vi "CRYO_MASTER_temp.vi"() -> ()   [LabVIEW 2017]
uses:
  LSI218Data.lvclass
  LSI336Data.lvclass
  USBData.lvclass
  <vilib>/Analysis/3filter.llb/FIR Filter (DBL).vi
  <vilib>/DAQmx/create/channels.llb/DAQmx Create Channel (DO-Digital Output).vi
  <vilib>/DAQmx/miscellaneous.llb/DAQmx Fill In Error Info.vi
  <vilib>/Analysis/NI_AALBase.lvlib
panel:
  out "Cycle #":u32=6
  in  "Measurement Interval (s)":dbl=1.0
  in  "Stop Button":bool
  in  "?":T1(tab)=enum."INPUT CONFIG 2"
  in  "Record interval (USB6218)":i64=10
  in  "InstName (USB6218)":string="USB6218"
  in  "USB6218 Config":T2(array[cluster])=[{"Label"="F_1", "FileFormat"="%5.5f", "Active?"=TRUE, "Physical CH"="Dev1/ai0", " terminal\n type"=10083, "ConversionType"={"Type"=enum."SimpleProp", "ConversionParameters"=[0.0, 5.0, 0.0, 500.0]}, "VoltageLimits"=[0.0, 5.0]}, {"Label"="F_2", "FileFormat"="%5.5f", "Active?"=TRUE, "Physical CH"="Dev1/ai1", " terminal\n type"=10083, "ConversionType"={"Type"=enum."SimpleProp", "ConversionParameters"=[0.0, 5.0, 0.0, 500.0]}, "VoltageLimits"=[0.0, 5.0]}, {"Label"="F_3", "FileFormat"="%5.5f", "Active?"=TRUE, "Physical CH"="Dev1/ai2", " terminal\n type"=10083, "ConversionType"={"Type"=enum."SimpleProp", "ConversionParameters"=[0.0, 5.0, 0.0, 500.0]}, "VoltageLimits"=[0.0, 5.0]}, {"Label"="F_4", "FileFormat"="%5.5f", "Active?"=TRUE, "Physical CH"="Dev1/ai3", " terminal\n type"=10083, "ConversionType"={"Type"=enum."SimpleProp", "ConversionParameters"=[0.0, 5.0, 0.0, 500.0]}, "VoltageLimits"=[0.0, 5.0]}, {"Label"="F_5", "FileFormat"="%5.5f", "Active?"=FALSE, "Physical CH"="Dev1/ai4", " terminal\n type"=10083, "ConversionType"={"Type"=enum."SimpleProp", "ConversionParameters"=[0.0, 5.0, 0.0, 500.0]}, "VoltageLimits"=[0.0, 6.0]}] {"terminal\n type" items=["Default"=-1, "RSE"=10083, "NRSE"=10078, "Differential"=10106, "Pseudodifferential"=12529]}
  out "error out (USB6218)":errorcluster={"status"=TRUE, "code"=-201426, "source"="DAQmx Start Task.vi:7220001<append>\n<B>Device: </B>Dev1\n<B>Device: </B>Dev2\n\n<B>Task Name: </B>NoiseCheck_20200908_163740_USB6218__AIN"}
  out "error out (USB6210/6218 DOUT)":errorcluster
  out "Target Index":i32=-1
  out "DOUT task out":refnum<k21>="20200908_153558_DO"
  in  "DOUT for Vavle V2 (N.C.)":tag="Dev1/port1/line1"
  in  "DOUT for Vavle V1 (N.O.)":tag="Dev1/port1/line0"
  in  "TargetSignal Label":string="P_Dewar"
  in  "Digital Out ON?":bool
  in  "Record interval (USB6210)":i64=10
  in  "USB6210 Config":T2(array[cluster])=[{"Label"="P_ins", "FileFormat"="%5.5e", "Active?"=TRUE, "Physical CH"="Dev2/ai0", " terminal\n type"=10083, "ConversionType"={"Type"=enum."CC-10_LOG", "ConversionParameters"=[0.5, 9.0, 0.0, 1.0]}, "VoltageLimits"=[0.0, 10.0]}, {"Label"="P_4Kres", "FileFormat"="%5.5e", "Active?"=TRUE, "Physical CH"="Dev2/ai1", " terminal\n type"=10083, "ConversionType"={"Type"=enum."SimpleProp", "ConversionParameters"=[1.0, 5.0, 0.0, 200000.0]}, "VoltageLimits"=[0.0, 5.0]}, {"Label"="P_3HeIN", "FileFormat"="%5.5e", "Active?"=TRUE, "Physical CH"="Dev2/ai2", " terminal\n type"=10083, "ConversionType"={"Type"=enum."SimpleProp", "ConversionParameters"=[1.0, 5.0, 0.0, 200000.0]}, "VoltageLimits"=[0.0, 5.0]}, {"Label"="P_SldRTN", "FileFormat"="%5.5e", "Active?"=TRUE, "Physical CH"="Dev2/ai3", " terminal\n type"=10083, "ConversionType"={"Type"=enum."SimpleProp", "ConversionParameters"=[1.0, 5.0, 0.0, 200000.0]}, "VoltageLimits"=[0.0, 5.0]}, {"Label"="P_3Hepot", "FileFormat"="%5.5e", "Active?"=TRUE, "Physical CH"="Dev2/ai4", " terminal\n type"=10083, "ConversionType"={"Type"=enum."SimpleProp", "ConversionParameters"=[0.0, 10.0, 0.0, 133320.0]}, "VoltageLimits"=[0.0, 10.0]}, {"Label"="P_1Kepot", "FileFormat"="%5.5e", "Active?"=TRUE, "Physical CH"="Dev2/ai5", " terminal\n type"=10083, "ConversionType"={"Type"=enum."SimpleProp", "ConversionParameters"=[0.0, 10.0, 0.0, 133320.0]}, "VoltageLimits"=[0.0, 10.0]}, {"Label"="P_Dewar", "FileFormat"="%5.5e", "Active?"=TRUE, "Physical CH"="Dev2/ai6", " terminal\n type"=10083, "ConversionType"={"Type"=enum."SimpleProp", "ConversionParameters"=[1.0, 5.0, 0.0, 200000.0]}, "VoltageLimits"=[0.0, 5.0]}, {"Label"="DP_HEX4", "FileFormat"="%5.5e", "Active?"=TRUE, "Physical CH"="Dev2/ai7", " terminal\n type"=10083, "ConversionType"={"Type"=enum."SimpleProp", "ConversionParameters"=[1.0, 5.0, 0.0, 20000.0]}, "VoltageLimits"=[0.0, 5.0]}, {"Label"="DP_HEX5", "FileFormat"="%5.5e", "Active?"=TRUE, "Physical CH"="Dev2/ai8", " terminal\n type"=10083, "ConversionType"={"Type"=enum."SimpleProp", "ConversionParameters"=[1.0, 5.0, 0.0, 20000.0]}, "VoltageLimits"=[0.0, 5.0]}, {"Label"="L1", "FileFormat"="%5.5f", "Active?"=TRUE, "Physical CH"="Dev2/ai9", " terminal\n type"=10083, "ConversionType"={"Type"=enum."SimpleProp", "ConversionParameters"=[0.0, 10.0, 0.0, 100.0]}, "VoltageLimits"=[0.0, 10.0]}, {"Label"="L2-1", "FileFormat"="%5.5f", "Active?"=TRUE, "Physical CH"="Dev2/ai10", " terminal\n type"=10083, "ConversionType"={"Type"=enum."SimpleProp", "ConversionParameters"=[0.0, 10.0, 0.0, 100.0]}, "VoltageLimits"=[0.0, 10.0]}, {"Label"="L2-2", "FileFormat"="%5.5f", "Active?"=TRUE, "Physical CH"="Dev2/ai11", " terminal\n type"=10083, "ConversionType"={"Type"=enum."SimpleProp", "ConversionParameters"=[0.0, 10.0, 0.0, 100.0]}, "VoltageLimits"=[0.0, 10.0]}, {"Label"="L3", "FileFormat"="%5.5f", "Active?"=TRUE, "Physical CH"="Dev2/ai12", " terminal\n type"=10083, "ConversionType"={"Type"=enum."SimpleProp", "ConversionParameters"=[0.0, 10.0, 0.0, 100.0]}, "VoltageLimits"=[0.0, 10.0]}] {"terminal\n type" items=["Default"=-1, "RSE"=10083, "NRSE"=10078, "Differential"=10106, "Pseudodifferential"=12529]}
  in  "RUN identifier":string="MeasureBuildup"
  in  "Base Path":path=path "C:/LabVIEW/DATA/Precooling"
  in  "InstName (USB6210)":string="USB6210"
  out "error out (USB6210)":errorcluster
  in  "Record interval (LSI336)":i64=10
  in  "Record interval (LSI218)":i64=10
  out "error out (LSI336)":errorcluster
  in  "InstName (LSI336)":string="LSI336"
  in  "FileFormat (336)":string="%4.4f"
  in  "LSI336Settings(X,Y)":T3(array[cluster])=[{"LSIName"="LSi336X", "Labels"=["T1K3-1", "T1K3-2", "T3He5", "T3He8"], "SensorLocations"=[enum."T1K3-1", enum."T1K3-2", enum."T3He5", enum."T3He8"], "Active?"=TRUE, "VISA res. name"="GPIB0::1::INSTR"}, {"LSIName"="LSi336Y", "Labels"=["T3He6-1", "T3He6-2", "T3He7-1", "T3He7-2"], "SensorLocations"=[enum."T3He6-1", enum."T3He6-2", enum."T3He7-1", enum."T3He7-2"], "Active?"=TRUE, "VISA res. name"="GPIB0::2::INSTR"}]
  in  "FileFormat (218)":string="%4.4f"
  in  "InstName (LSI218)":string="LSI218"
  in  "LSI218Settings(A-F)":T3(array[cluster])=[{"LSIName"="LSI218A", "Labels"=["T3He10", "T3He1-1", "TTH3", "TTH4", "TTH1", "TTH2", "T4He1", "T1K1"], "SensorLocations"=[enum."T3He10", enum."T3He1-1", enum."TTH3", enum."TTH4", enum."TTH1", enum."TTH2", enum."T4He1", enum."T1K1"], "Active?"=TRUE, "VISA res. name"="GPIB0::7::INSTR"}, {"LSIName"="LSI218B", "Labels"=["N.C.", "N.C.", "N.C.", "N.C.", "T3He2-1", "T3He2-2", "T3He3", "T3He1-4"], "SensorLocations"=[enum."N.C.", enum."N.C.", enum."N.C.", enum."T3He1-4", enum."T3He2-1", enum."T3He2-2", enum."T3He3", enum."T3He1-4"], "Active?"=TRUE, "VISA res. name"="GPIB0::4::INSTR"}, {"LSIName"="LSI218C", "Labels"=["T4He3-1", "T4He3-2", "T4He3-3", "T4He3-4", "T4He2-1", "T4He2-2", "T4He4", "T4He5"], "SensorLocations"=[enum."T4He3-1", enum."T4He3-2", enum."T4He3-3", enum."T4He3-4", enum."T4He2-1", enum."T4He2-2", enum."T4He4", enum."T4He5"], "Active?"=TRUE, "VISA res. name"="GPIB0::3::INSTR"}, {"LSIName"="LSI218D", "Labels"=["T4He6", "T4He9", "T3He1-2", "T3He1-3", "T4He7", "T4He8", "T4He10", "T1K6"], "SensorLocations"=[enum."T4He6", enum."T4He9", enum."T3He1-2", enum."T3He1-3", enum."T4He7", enum."T4He8", enum."T4He10", enum."T1K6"], "Active?"=TRUE, "VISA res. name"="GPIB0::5::INSTR"}, {"LSIName"="LSI218E", "Labels"=["TIP1", "N.C.", "TIP2", "N.C.", "TIP3", "TIP4", "TIP5", "N.C."], "SensorLocations"=[enum."TIP1", enum."N.C.", enum."TIP2", enum."N.C.", enum."TIP3", enum."TIP4", enum."TIP5", enum."N.C."], "Active?"=TRUE, "VISA res. name"="GPIB0::11::INSTR"}, {"LSIName"="LSI218F", "Labels"=["T1K2", "T1K4", "T1K5", "T3He4", "T3He9", "TIP6", "N.C.", "N.C."], "SensorLocations"=[enum."T1K2", enum."T1K4", enum."T1K5", enum."T3He4", enum."T3He9", enum."TIP6", enum."N.C.", enum."N.C."], "Active?"=TRUE, "VISA res. name"="GPIB0::8::INSTR"}]
  out "error out (LSI218)":errorcluster
  in  "FIle suffix 4":string="Graph4"
  in  "Take Screenshot! 4":bool
  in  "FIle suffix 3":string="Graph3"
  in  "Take Screenshot! 3":bool
  in  "FIle suffix 2":string="Graph2"
  in  "Take Screenshot! 2":bool
  in  "FIle suffix 1":string="Graph1"
  in  "Take Screenshot! 1":bool
  in  "log/linear 2":bool
  in  "Tab Control 2":T4(tab)=enum."USB6218"
  in  "Plot selecter (USB6210)\n    1      2     3     4":bool[][](array[boolean])=[[FALSE, FALSE, TRUE, FALSE], [FALSE, FALSE, TRUE, FALSE], [FALSE, FALSE, TRUE, FALSE], [FALSE, FALSE, TRUE, FALSE], [FALSE, FALSE, TRUE, FALSE], [FALSE, FALSE, TRUE, FALSE], [TRUE, FALSE, FALSE, FALSE], [FALSE, FALSE, TRUE, FALSE], [FALSE, FALSE, TRUE, FALSE], [FALSE, FALSE, FALSE, TRUE], [FALSE, FALSE, FALSE, TRUE], [FALSE, FALSE, FALSE, TRUE], [FALSE, FALSE, FALSE, TRUE], [FALSE, FALSE, FALSE, FALSE], [FALSE, FALSE, FALSE, FALSE], [FALSE, FALSE, FALSE, FALSE]]
  out "All Labels (USB6210)":string[](array[string])=["P_ins", "P_4Kres", "P_3HeIN", "P_SldRTN", "P_3Hepot", "P_1Kepot", "P_Dewar", "DP_HEX4", "DP_HEX5", "L1", "L2-1", "L2-2", "L3"]
  out "Last Data \n(USB6210)":dbl[](array[numeric])=[0.0010673459546745845, 101235.2421096093, 101172.75380845381, 101180.97599727615, 331.5883530972572, 77.33204658868218, 101532.88361704744, -4900.627465235827, -39.11406425463837, 99.96245786292866, 0.020520200367966923, 0.23227550766425742, 100.52409354456952] format="%#_6e"
  out "Time of Last Measurement (USB6210)":timestamp=timestamp(3682395466.7858553 s since 1904-01-01)
  out "USB6210 Status":T5(ring)=enum."Ready"
  out "Last Vol\n(USB6210)":dbl[](array[numeric])=[6.014152604208098, 3.024704842192186, 3.023455076169076, 3.023619519945523, 0.024871613643658655, 0.005800483542505413, 3.030657672340949, 0.01987450695283468, 0.9921771871490723, 9.996245786292866, 0.0020520200367966923, 0.023227550766425742, 10.052409354456952] format="%_5f"
  out "Time of Last Measurement (USB6218)":timestamp
  out "USB6218 Status":T5(ring)=enum."Ready"
  out "Last Vol \n(USB6218)":dbl[](array[numeric]) format="%_5f"
  out "Last Data \n(USB6218)":dbl[](array[numeric]) format="%#_6e"
  out "All Labels (USB6218)":string[](array[string])
  in  "Plot selecter (USB6218)\n    1      2     3     5":bool[][](array[boolean])=[[FALSE, FALSE, TRUE, FALSE], [FALSE, FALSE, TRUE, FALSE], [FALSE, FALSE, TRUE, FALSE], [FALSE, FALSE, TRUE, FALSE], [FALSE, FALSE, TRUE, FALSE], [FALSE, FALSE, TRUE, FALSE], [TRUE, FALSE, FALSE, FALSE], [FALSE, FALSE, TRUE, FALSE], [FALSE, FALSE, TRUE, FALSE], [FALSE, FALSE, FALSE, TRUE], [FALSE, FALSE, FALSE, TRUE], [FALSE, FALSE, FALSE, TRUE], [FALSE, FALSE, FALSE, TRUE], [FALSE, FALSE, FALSE, FALSE], [FALSE, FALSE, FALSE, FALSE], [FALSE, FALSE, FALSE, FALSE]]
  out "Time of Last Measurement (LSI218)":timestamp=timestamp(3682395466.7858553 s since 1904-01-01)
  out "LSI218 Status":T6(ring)=enum."Measuring"
  out "Last Data \nLSI218 (1)":dbl[](array[numeric])=[297.17, 297.3, 296.26, 296.72, 295.15, 295.39, 294.82, 294.9, 30.0, 0.0, 0.0, 0.0, 296.0, 296.28, 295.4, 296.77, 296.94, 297.1, 296.87, 296.9, 295.77, 295.79, 295.93, 295.83]
  out "Labels LSI218 (1)":string[](array[string])=["T3He10", "T3He1-1", "TTH3", "TTH4", "TTH1", "TTH2", "T4He1", "T1K1", "N.C.", "N.C.", "N.C.", "N.C.", "T3He2-1", "T3He2-2", "T3He3", "T3He1-4", "T4He3-1", "T4He3-2", "T4He3-3", "T4He3-4", "T4He2-1", "T4He2-2", "T4He4", "T4He5"]
  in  "Plot selecter LSI218(1)\n    1      2     3     4":bool[][](array[boolean])=[[FALSE, FALSE, FALSE, FALSE], [FALSE, FALSE, FALSE, FALSE], [FALSE, FALSE, FALSE, FALSE], [FALSE, FALSE, FALSE, FALSE], [FALSE, FALSE, FALSE, FALSE], [FALSE, FALSE, FALSE, FALSE], [FALSE, FALSE, FALSE, FALSE], [FALSE, FALSE, FALSE, FALSE], [FALSE, FALSE, FALSE, FALSE], [FALSE, FALSE, FALSE, FALSE], [FALSE, FALSE, FALSE, FALSE], [FALSE, FALSE, FALSE, FALSE], [FALSE, FALSE, FALSE, FALSE], [FALSE, FALSE, FALSE, FALSE], [FALSE, FALSE, FALSE, FALSE], [FALSE, FALSE, FALSE, FALSE], [FALSE, FALSE, FALSE, FALSE], [FALSE, FALSE, FALSE, FALSE], [FALSE, FALSE, FALSE, FALSE], [FALSE, FALSE, FALSE, FALSE], [FALSE, FALSE, FALSE, FALSE], [FALSE, FALSE, FALSE, FALSE], [FALSE, FALSE, FALSE, FALSE], [FALSE, FALSE, FALSE, FALSE]]
  out "Active?\n (1)":bool[](array[boolean])=[TRUE, TRUE, TRUE, TRUE, TRUE, TRUE, TRUE, TRUE, TRUE, TRUE, TRUE, TRUE, TRUE, TRUE, TRUE, TRUE, TRUE, TRUE, TRUE, TRUE, TRUE, TRUE, TRUE, TRUE]
  out "Labels LSI218 (2)":string[](array[string])=["T4He6", "T4He9", "T3He1-2", "T3He1-3", "T4He7", "T4He8", "T4He10", "T1K6", "TIP1", "N.C.", "TIP2", "N.C.", "TIP3", "TIP4", "TIP5", "N.C.", "T1K2", "T1K4", "T1K5", "T3He4", "T3He9", "TIP6", "N.C.", "N.C."]
  out "Active?\n(2)":bool[](array[boolean])=[TRUE, TRUE, TRUE, TRUE, TRUE, TRUE, TRUE, TRUE, TRUE, TRUE, TRUE, TRUE, TRUE, TRUE, TRUE, TRUE, TRUE, TRUE, TRUE, TRUE, TRUE, TRUE, TRUE, TRUE]
  out "Last Data \nLSI218 (2)":dbl[](array[numeric])=[296.1, 296.73, 297.5, 297.11, 296.33, 296.83, 296.68, 296.96, 296.62, 0.0, 295.89, 688.49, 295.65, 295.44, 295.46, 688.58, 300.85, 297.13, 297.64, 294.64, 288.62, 287.47, 0.433, 0.0]
  in  "Plot selecter LSI218(2)\n    1      2     3     4":bool[][](array[boolean])=[[FALSE, TRUE, FALSE, FALSE], [FALSE, TRUE, FALSE, FALSE], [FALSE, TRUE, FALSE, FALSE], [FALSE, TRUE, FALSE, FALSE], [FALSE, TRUE, FALSE, FALSE], [FALSE, TRUE, FALSE, FALSE], [FALSE, TRUE, FALSE, FALSE], [FALSE, TRUE, FALSE, FALSE], [FALSE, TRUE, FALSE, FALSE], [FALSE, TRUE, FALSE, FALSE], [FALSE, TRUE, FALSE, FALSE], [FALSE, FALSE, FALSE, FALSE], [FALSE, FALSE, FALSE, FALSE], [FALSE, FALSE, FALSE, FALSE], [FALSE, FALSE, FALSE, FALSE], [FALSE, FALSE, FALSE, FALSE], [FALSE, FALSE, FALSE, FALSE], [FALSE, FALSE, FALSE, FALSE], [FALSE, FALSE, FALSE, FALSE], [FALSE, FALSE, FALSE, FALSE], [FALSE, FALSE, FALSE, FALSE], [FALSE, FALSE, FALSE, FALSE], [FALSE, FALSE, FALSE, FALSE], [FALSE, FALSE, FALSE, FALSE]]
  in  "Plot selecter LSI336 \n     1      2     3     4":bool[][](array[boolean])=[[FALSE, TRUE, FALSE, FALSE], [FALSE, TRUE, FALSE, FALSE], [FALSE, TRUE, FALSE, FALSE], [FALSE, TRUE, FALSE, FALSE], [FALSE, TRUE, FALSE, FALSE], [FALSE, TRUE, FALSE, FALSE], [FALSE, TRUE, FALSE, FALSE], [FALSE, TRUE, FALSE, FALSE]]
  out "Time of Last Measurement (LSI336) 2":timestamp=timestamp(3682395466.7858553 s since 1904-01-01)
  out "Last Data \nLSI336":dbl[](array[numeric])=[295.892, 295.621, 295.543, 295.514, 295.418, 295.377, 295.467, 295.916]
  out "Active?\n(LSI336)":bool[](array[boolean])=[TRUE, TRUE, TRUE, TRUE, TRUE, TRUE, TRUE, TRUE]
  out "Labels LSI336":string[](array[string])=["T1K3-1", "T1K3-2", "T3He5", "T3He8", "T3He6-1", "T3He6-2", "T3He7-1", "T3He7-2"]
  out "LSI336 Status":T6(ring)=enum."Measuring"
  out "Graph 1":T7(graph)=[{"TimeArray"=[timestamp(3682395461.78455 s since 1904-01-01), timestamp(3682395462.7856207 s since 1904-01-01), timestamp(3682395463.785891 s since 1904-01-01), timestamp(3682395464.7859097 s since 1904-01-01), timestamp(3682395465.7859406 s since 1904-01-01), timestamp(3682395466.7858553 s since 1904-01-01)], "LDArray"=[101513.15068695585]}] caption="XY Graph"
  in  "log/linear 1":bool
  out "Graph 2":T8(graph)=[{"TimeArray"=[timestamp(3682395461.78455 s since 1904-01-01), timestamp(3682395462.7856207 s since 1904-01-01), timestamp(3682395463.785891 s since 1904-01-01), timestamp(3682395464.7859097 s since 1904-01-01), timestamp(3682395465.7859406 s since 1904-01-01), timestamp(3682395466.7858553 s since 1904-01-01)], "DataArray"=[296.06, 296.09, 296.09, 296.05, 296.06, 296.1]}, {"TimeArray"=[timestamp(3682395461.78455 s since 1904-01-01), timestamp(3682395462.7856207 s since 1904-01-01), timestamp(3682395463.785891 s since 1904-01-01), timestamp(3682395464.7859097 s since 1904-01-01), timestamp(3682395465.7859406 s since 1904-01-01), timestamp(3682395466.7858553 s since 1904-01-01)], "DataArray"=[296.71, 296.73, 296.74, 296.71, 296.73, 296.73]}, {"TimeArray"=[timestamp(3682395461.78455 s since 1904-01-01), timestamp(3682395462.7856207 s since 1904-01-01), timestamp(3682395463.785891 s since 1904-01-01), timestamp(3682395464.7859097 s since 1904-01-01), timestamp(3682395465.7859406 s since 1904-01-01), timestamp(3682395466.7858553 s since 1904-01-01)], "DataArray"=[297.47, 297.49, 297.49, 297.49, 297.49, 297.5]}, {"TimeArray"=[timestamp(3682395461.78455 s since 1904-01-01), timestamp(3682395462.7856207 s since 1904-01-01), timestamp(3682395463.785891 s since 1904-01-01), timestamp(3682395464.7859097 s since 1904-01-01), timestamp(3682395465.7859406 s since 1904-01-01), timestamp(3682395466.7858553 s since 1904-01-01)], "DataArray"=[297.12, 297.1, 297.1, 297.12, 297.11, 297.11]}, {"TimeArray"=[timestamp(3682395461.78455 s since 1904-01-01), timestamp(3682395462.7856207 s since 1904-01-01), timestamp(3682395463.785891 s since 1904-01-01), timestamp(3682395464.7859097 s since 1904-01-01), timestamp(3682395465.7859406 s since 1904-01-01), timestamp(3682395466.7858553 s since 1904-01-01)], "DataArray"=[296.31, 296.33, 296.32, 296.3, 296.32, 296.33]}, {"TimeArray"=[timestamp(3682395461.78455 s since 1904-01-01), timestamp(3682395462.7856207 s since 1904-01-01), timestamp(3682395463.785891 s since 1904-01-01), timestamp(3682395464.7859097 s since 1904-01-01), timestamp(3682395465.7859406 s since 1904-01-01), timestamp(3682395466.7858553 s since 1904-01-01)], "DataArray"=[296.84, 296.82, 296.85, 296.82, 296.83, 296.83]}, {"TimeArray"=[timestamp(3682395461.78455 s since 1904-01-01), timestamp(3682395462.7856207 s since 1904-01-01), timestamp(3682395463.785891 s since 1904-01-01), timestamp(3682395464.7859097 s since 1904-01-01), timestamp(3682395465.7859406 s since 1904-01-01), timestamp(3682395466.7858553 s since 1904-01-01)], "DataArray"=[296.68, 296.7, 296.7, 296.71, 296.7, 296.68]}, {"TimeArray"=[timestamp(3682395461.78455 s since 1904-01-01), timestamp(3682395462.7856207 s since 1904-01-01), timestamp(3682395463.785891 s since 1904-01-01), timestamp(3682395464.7859097 s since 1904-01-01), timestamp(3682395465.7859406 s since 1904-01-01), timestamp(3682395466.7858553 s since 1904-01-01)], "DataArray"=[296.95, 296.97, 296.97, 296.96, 296.96, 296.96]}, {"TimeArray"=[timestamp(3682395461.78455 s since 1904-01-01), timestamp(3682395462.7856207 s since 1904-01-01), timestamp(3682395463.785891 s since 1904-01-01), timestamp(3682395464.7859097 s since 1904-01-01), timestamp(3682395465.7859406 s since 1904-01-01), timestamp(3682395466.7858553 s since 1904-01-01)], "DataArray"=[296.61, 296.61, 296.62, 296.62, 296.62, 296.62]}, {"TimeArray"=[timestamp(3682395461.78455 s since 1904-01-01), timestamp(3682395462.7856207 s since 1904-01-01), timestamp(3682395463.785891 s since 1904-01-01), timestamp(3682395464.7859097 s since 1904-01-01), timestamp(3682395465.7859406 s since 1904-01-01), timestamp(3682395466.7858553 s since 1904-01-01)], "DataArray"=[0.0, 0.0, 0.0, 0.0, 0.0, 0.0]}, {"TimeArray"=[timestamp(3682395461.78455 s since 1904-01-01), timestamp(3682395462.7856207 s since 1904-01-01), timestamp(3682395463.785891 s since 1904-01-01), timestamp(3682395464.7859097 s since 1904-01-01), timestamp(3682395465.7859406 s since 1904-01-01), timestamp(3682395466.7858553 s since 1904-01-01)], "DataArray"=[295.89, 295.9, 295.89, 295.89, 295.89, 295.89]}, {"TimeArray"=[timestamp(3682395461.78455 s since 1904-01-01), timestamp(3682395462.7856207 s since 1904-01-01), timestamp(3682395463.785891 s since 1904-01-01), timestamp(3682395464.7859097 s since 1904-01-01), timestamp(3682395465.7859406 s since 1904-01-01), timestamp(3682395466.7858553 s since 1904-01-01)], "DataArray"=[295.88, 295.884, 295.883, 295.878, 295.892, 295.892]}, {"TimeArray"=[timestamp(3682395461.78455 s since 1904-01-01), timestamp(3682395462.7856207 s since 1904-01-01), timestamp(3682395463.785891 s since 1904-01-01), timestamp(3682395464.7859097 s since 1904-01-01), timestamp(3682395465.7859406 s since 1904-01-01), timestamp(3682395466.7858553 s since 1904-01-01)], "DataArray"=[295.635, 295.636, 295.626, 295.624, 295.627, 295.621]}, {"TimeArray"=[timestamp(3682395461.78455 s since 1904-01-01), timestamp(3682395462.7856207 s since 1904-01-01), timestamp(3682395463.785891 s since 1904-01-01), timestamp(3682395464.7859097 s since 1904-01-01), timestamp(3682395465.7859406 s since 1904-01-01), timestamp(3682395466.7858553 s since 1904-01-01)], "DataArray"=[295.548, 295.536, 295.543, 295.551, 295.548, 295.543]}, {"TimeArray"=[timestamp(3682395461.78455 s since 1904-01-01), timestamp(3682395462.7856207 s since 1904-01-01), timestamp(3682395463.785891 s since 1904-01-01), timestamp(3682395464.7859097 s since 1904-01-01), timestamp(3682395465.7859406 s since 1904-01-01), timestamp(3682395466.7858553 s since 1904-01-01)], "DataArray"=[295.512, 295.511, 295.514, 295.494, 295.506, 295.514]}, {"TimeArray"=[timestamp(3682395461.78455 s since 1904-01-01), timestamp(3682395462.7856207 s since 1904-01-01), timestamp(3682395463.785891 s since 1904-01-01), timestamp(3682395464.7859097 s since 1904-01-01), timestamp(3682395465.7859406 s since 1904-01-01), timestamp(3682395466.7858553 s since 1904-01-01)], "DataArray"=[295.413, 295.428, 295.418, 295.414, 295.415, 295.418]}, {"TimeArray"=[timestamp(3682395461.78455 s since 1904-01-01), timestamp(3682395462.7856207 s since 1904-01-01), timestamp(3682395463.785891 s since 1904-01-01), timestamp(3682395464.7859097 s since 1904-01-01), timestamp(3682395465.7859406 s since 1904-01-01), timestamp(3682395466.7858553 s since 1904-01-01)], "DataArray"=[295.383, 295.374, 295.388, 295.38, 295.372, 295.377]}, {"TimeArray"=[timestamp(3682395461.78455 s since 1904-01-01), timestamp(3682395462.7856207 s since 1904-01-01), timestamp(3682395463.785891 s since 1904-01-01), timestamp(3682395464.7859097 s since 1904-01-01), timestamp(3682395465.7859406 s since 1904-01-01), timestamp(3682395466.7858553 s since 1904-01-01)], "DataArray"=[295.453, 295.444, 295.449, 295.458, 295.449, 295.467]}, {"TimeArray"=[timestamp(3682395461.78455 s since 1904-01-01), timestamp(3682395462.7856207 s since 1904-01-01), timestamp(3682395463.785891 s since 1904-01-01), timestamp(3682395464.7859097 s since 1904-01-01), timestamp(3682395465.7859406 s since 1904-01-01), timestamp(3682395466.7858553 s since 1904-01-01)], "DataArray"=[295.913, 295.896, 295.909, 295.904, 295.905, 295.916]}] caption="XY Graph"
  out "Graph 3":T8(graph)=[{"TimeArray"=[timestamp(3682395461.78455 s since 1904-01-01), timestamp(3682395462.7856207 s since 1904-01-01), timestamp(3682395463.785891 s since 1904-01-01), timestamp(3682395464.7859097 s since 1904-01-01), timestamp(3682395465.7859406 s since 1904-01-01), timestamp(3682395466.7858553 s since 1904-01-01)], "DataArray"=[0.0010323744543872916]}, {"TimeArray"=[timestamp(3682395461.78455 s since 1904-01-01), timestamp(3682395462.7856207 s since 1904-01-01), timestamp(3682395463.785891 s since 1904-01-01), timestamp(3682395464.7859097 s since 1904-01-01), timestamp(3682395465.7859406 s since 1904-01-01), timestamp(3682395466.7858553 s since 1904-01-01)], "DataArray"=[100727.11432139605]}, {"TimeArray"=[timestamp(3682395461.78455 s since 1904-01-01), timestamp(3682395462.7856207 s since 1904-01-01), timestamp(3682395463.785891 s since 1904-01-01), timestamp(3682395464.7859097 s since 1904-01-01), timestamp(3682395465.7859406 s since 1904-01-01), timestamp(3682395466.7858553 s since 1904-01-01)], "DataArray"=[101228.66431734736]}, {"TimeArray"=[timestamp(3682395461.78455 s since 1904-01-01), timestamp(3682395462.7856207 s since 1904-01-01), timestamp(3682395463.785891 s since 1904-01-01), timestamp(3682395464.7859097 s since 1904-01-01), timestamp(3682395465.7859406 s since 1904-01-01), timestamp(3682395466.7858553 s since 1904-01-01)], "DataArray"=[101455.59517360969]}, {"TimeArray"=[timestamp(3682395461.78455 s since 1904-01-01), timestamp(3682395462.7856207 s since 1904-01-01), timestamp(3682395463.785891 s since 1904-01-01), timestamp(3682395464.7859097 s since 1904-01-01), timestamp(3682395465.7859406 s since 1904-01-01), timestamp(3682395466.7858553 s since 1904-01-01)], "DataArray"=[363.15120439796374]}, {"TimeArray"=[timestamp(3682395461.78455 s since 1904-01-01), timestamp(3682395462.7856207 s since 1904-01-01), timestamp(3682395463.785891 s since 1904-01-01), timestamp(3682395464.7859097 s since 1904-01-01), timestamp(3682395465.7859406 s since 1904-01-01), timestamp(3682395466.7858553 s since 1904-01-01)], "DataArray"=[-31.38444278817984]}, {"TimeArray"=[timestamp(3682395461.78455 s since 1904-01-01), timestamp(3682395462.7856207 s since 1904-01-01), timestamp(3682395463.785891 s since 1904-01-01), timestamp(3682395464.7859097 s since 1904-01-01), timestamp(3682395465.7859406 s since 1904-01-01), timestamp(3682395466.7858553 s since 1904-01-01)], "DataArray"=[-4917.400374415536]}, {"TimeArray"=[timestamp(3682395461.78455 s since 1904-01-01), timestamp(3682395462.7856207 s since 1904-01-01), timestamp(3682395463.785891 s since 1904-01-01), timestamp(3682395464.7859097 s since 1904-01-01), timestamp(3682395465.7859406 s since 1904-01-01), timestamp(3682395466.7858553 s since 1904-01-01)], "DataArray"=[-75.78428391488757]}] caption="XY Graph"
  out "Graph 4":T8(graph)=[{"TimeArray"=[timestamp(3682395461.78455 s since 1904-01-01), timestamp(3682395462.7856207 s since 1904-01-01), timestamp(3682395463.785891 s since 1904-01-01), timestamp(3682395464.7859097 s since 1904-01-01), timestamp(3682395465.7859406 s since 1904-01-01), timestamp(3682395466.7858553 s since 1904-01-01)], "DataArray"=[100.06965528297283]}, {"TimeArray"=[timestamp(3682395461.78455 s since 1904-01-01), timestamp(3682395462.7856207 s since 1904-01-01), timestamp(3682395463.785891 s since 1904-01-01), timestamp(3682395464.7859097 s since 1904-01-01), timestamp(3682395465.7859406 s since 1904-01-01), timestamp(3682395466.7858553 s since 1904-01-01)], "DataArray"=[0.09285897020154232]}, {"TimeArray"=[timestamp(3682395461.78455 s since 1904-01-01), timestamp(3682395462.7856207 s since 1904-01-01), timestamp(3682395463.785891 s since 1904-01-01), timestamp(3682395464.7859097 s since 1904-01-01), timestamp(3682395465.7859406 s since 1904-01-01), timestamp(3682395466.7858553 s since 1904-01-01)], "DataArray"=[0.10601147435317196]}, {"TimeArray"=[timestamp(3682395461.78455 s since 1904-01-01), timestamp(3682395462.7856207 s since 1904-01-01), timestamp(3682395463.785891 s since 1904-01-01), timestamp(3682395464.7859097 s since 1904-01-01), timestamp(3682395465.7859406 s since 1904-01-01), timestamp(3682395466.7858553 s since 1904-01-01)], "DataArray"=[100.57867875758531]}] caption="XY Graph"
  in  "log/linear 4":bool
  in  "log/linear 3":bool
  in  "P_safelimit_up (Pa)":dbl=5000.0 format="%_4e"
  in  "P_safelimit_low (Pa)":dbl=5000.0 format="%_4e"
  out "Pav - (P_2_th_high+P_2_tol)=":dbl
  in  "Auto ON?":bool
  out "Pstd history":dbl(graph)=554.7391446242465
  out "Pav history":dbl(graph)=-49199.19854911039
  in  "Mov. Avg Interval":i64=4
  in  "V2 (N.C.)":bool
  in  "V1 (N.O.)":bool=TRUE
  in  "N for sampling":i64=7
  in  "P_2_tol (Pa)":dbl=5000.0 format="%_4e"
  in  "P_1_tol (Pa)":dbl=5000.0 format="%_4e"
  in  "P_2_th_low (Pa)":dbl=125000.0 format="%_4e"
  in  "P_1_th_low (Pa)":dbl=125000.0 format="%_4g"
  in  "P_2_th_high (Pa)":dbl=130000.0 format="%_4e"
  in  "P_1_th_high (Pa)":dbl=130000.0 format="%_4e"
  out "Graph 5":T9(graph) caption="XY Graph"
  out "Last N M.A. Pressures":dbl[](array[numeric]) format="%_5e"
  out "Pav":dbl=-49199.19854911039 format="%0.4e"
  out "Pstd":dbl=554.7391446242465 format="%0.4e"
  out "Status V2 CTRL":enum16{"Pressurize", "Depressurize"}(ring)
  out "Status V1 CTRL":enum16{"Pressurize", "Depressurize"}(ring)
  out "Pav - (P_2_th_low_-P_2_tol)=":dbl
  out "Pav - (P_1_th_low_-P_1_tol)=":dbl
  out "Pav - (P_1_th_high+P_1_tol)=":dbl
  out "Series 1":string[](array[string])=["P_Dewar"]
  out "Series 2":string[](array[string])=["T4He6", "T4He9", "T3He1-2", "T3He1-3", "T4He7", "T4He8", "T4He10", "T1K6", "TIP1", "N.C.", "TIP2", "T1K3-1", "T1K3-2", "T3He5", "T3He8", "T3He6-1", "T3He6-2", "T3He7-1", "T3He7-2"]
  out "Series 3":string[](array[string])=["P_ins", "P_4Kres", "P_3HeIN", "P_SldRTN", "P_3Hepot", "P_1Kepot", "DP_HEX4", "DP_HEX5"]
  out "Series 4":string[](array[string])=["L1", "L2-1", "L2-2", "L3"]
  out "Plot errors":errorcluster
  out "LastMeasurementConfig (218)":T10(array[cluster])=[{"LSIName"="LSI218A", "Active?"=TRUE, "LastData"=[297.17, 297.3, 296.26, 296.72, 295.15, 295.39, 294.82, 294.9], "Labels"=["T3He10", "T3He1-1", "TTH3", "TTH4", "TTH1", "TTH2", "T4He1", "T1K1"]}, {"LSIName"="LSI218B", "Active?"=TRUE, "LastData"=[30.0, 0.0, 0.0, 0.0, 296.0, 296.28, 295.4, 296.77], "Labels"=["N.C.", "N.C.", "N.C.", "N.C.", "T3He2-1", "T3He2-2", "T3He3", "T3He1-4"]}, {"LSIName"="LSI218C", "Active?"=TRUE, "LastData"=[296.94, 297.1, 296.87, 296.9, 295.77, 295.79, 295.93, 295.83], "Labels"=["T4He3-1", "T4He3-2", "T4He3-3", "T4He3-4", "T4He2-1", "T4He2-2", "T4He4", "T4He5"]}, {"LSIName"="LSI218D", "Active?"=TRUE, "LastData"=[296.1, 296.73, 297.5, 297.11, 296.33, 296.83, 296.68, 296.96], "Labels"=["T4He6", "T4He9", "T3He1-2", "T3He1-3", "T4He7", "T4He8", "T4He10", "T1K6"]}, {"LSIName"="LSI218E", "Active?"=TRUE, "LastData"=[296.62, 0.0, 295.89, 688.49, 295.65, 295.44, 295.46, 688.58], "Labels"=["TIP1", "N.C.", "TIP2", "N.C.", "TIP3", "TIP4", "TIP5", "N.C."]}, {"LSIName"="LSI218F", "Active?"=TRUE, "LastData"=[300.85, 297.13, 297.64, 294.64, 288.62, 287.47, 0.433, 0.0], "Labels"=["T1K2", "T1K4", "T1K5", "T3He4", "T3He9", "TIP6", "N.C.", "N.C."]}]
  out "DataArrayConv (USB)":dbl[][](array[numeric])=[[0.0010323744543872916, 100727.11432139605, 101228.66431734736, 101455.59517360969, 363.15120439796374, -31.38444278817984, 101513.15068695585, -4917.400374415536, -75.78428391488757, 100.06965528297283, 0.09285897020154232, 0.10601147435317196, 100.57867875758531]]